vi "Dresden R2R Sputter 03.02.2018 IY24.vi"() -> ()   [LabVIEW 2009] (continued)
                                n32107 = local read "R Cmb Ch2 Step2 Coating Power Active"() -> (w36745:bool)
                                n32108 = local read "R Cmb Ch2 Step3 Coating Power Active"() -> (w36744:bool)
                                n32109 = local read "R Cmb Ch2 Step4 Coating Power Active"() -> (w36743:bool)
                                n32110 = local read "R Cmb Ch2 Step5 Coating Power Active"() -> (w36742:bool)
                                n32111 = Boolean To (0,1)(Boolean=w36746) -> (0, 1=w36741:i16)
                                n32112 = Boolean To (0,1)(Boolean=w36745) -> (0, 1=w36740:i16)
                                n32113 = Boolean To (0,1)(Boolean=w36744) -> (0, 1=w36739:i16)
                                n32114 = Boolean To (0,1)(Boolean=w36743) -> (0, 1=w36738:i16)
                                n32115 = Boolean To (0,1)(Boolean=w36742) -> (0, 1=w36737:i16)
                                n32116 = Compound Arithmetic op=ADD(w36741, w36740, w36739, w36738, w36737) -> (w36735:i16)
                                n32117 = local read "R Cmb Interval length"() -> (w36736:dbl)
                                n32118 = Wait (ms)(milliseconds to wait=u32 200) -> ()  [unwired: 1 out]
                                n32119 = Multiply(x=w36736, y=w36735) -> (x*y=w36734:dbl)
                                n32120 = local write "Total length"(w36734) -> ()
                                }
                                frame #2 {
                                n32121 = local write "Calculate 2"(TRUE ("Calculate_auto")) -> ()
                                }
                                frame #3 {
                                n32122 = local write "Roll_side_select"(enum32{"Left to Right", "Right to Left"}."Left to Right" ("Roll_side_select")) -> ()
                                }
                                frame #4 {
                                n32123 = Wait (ms)(milliseconds to wait=u32 100) -> ()  [unwired: 1 out]
                                n32124 = local write "Parameters_auto_set"(TRUE ("Parameters_auto_set")) -> ()
                                }
                                frame #5 {
                                n32125 = while {
                                i -> [w36755]
                                stop <- w36751 stop-if-true
                                n32126 = Wait Until Next ms Multiple(millisecond multiple=u32 300) -> ()  [unwired: 1 out]
                                n32127 = Greater?(x=w36755, y=100) -> (0:w36752:bool)
                                n32128 = local read "Parameters_auto_set"() -> (w36756:bool)
                                n32129 = case shown="True" w36756 {
                                tunnel: [TRUE FALSE] -> w36753
                                frame #0 {
                                }
                                frame #1 {
                                }
                                }
                                n32130 = Or(x=w36753, y=w36752) -> (x .or. y?=w36751:bool)
                                }
                                }
                                frame #6 {
                                n32131 = local read "R Tension Value"() -> (w36760:dbl)
                                n32132 = Wait (ms)(milliseconds to wait=u32 200) -> ()  [unwired: 1 out]
                                n32133 = local write "TC1_set_value"(w36760) -> ()
                                }
                                frame #7 {
                                n32134 = local write "TC1_auto_set"(TRUE ("TC1_auto_set")) -> ()
                                }
                                frame #8 {
                                w36764 = u16 2 items=["1", "2", "3", "4"] ("Target Chamber Sensor")
                                n32135 = local write "Target Chamber Sensor"(w36764) -> ()
                                n32136 = Wait (ms)(milliseconds to wait=u32 200) -> ()  [unwired: 1 out]
                                }
                                frame #9 {
                                n32137 = local read "Total length"() -> (w36765:dbl)
                                n32138 = local write "Region"(w36765) -> ()
                                }
                                frame #10 {
                                n32139 = local read "Semi"() -> (w36766:bool)
                                n32140 = case shown="False" w36766 {
                                frame #0 {
                                n32141 = stacked-sequence {
                                frame #0 {
                                # "Gas Flow"
                                n32142 = stacked-sequence {
                                frame #0 {
                                n32143 = local read "Semi"() -> (w36767:bool)
                                n32144 = case shown="False" w36767 {
                                frame #0 {
                                n32145 = stacked-sequence {
                                frame #0 {
                                n32146 = local read "Semi"() -> (w36768:bool)
                                n32147 = case shown="False" w36768 {
                                frame #0 {
                                n32148 = local read "R Argon Flow sccm"() -> (w36769:dbl)
                                n32149 = local write "Ar_sccm3_4"(w36769) -> ()
                                }
                                frame #1 {
                                }
                                }
                                }
                                frame #1 {
                                n32150 = local read "Semi"() -> (w36770:bool)
                                n32151 = case shown="False" w36770 {
                                frame #0 {
                                n32152 = local write "Mfc2_Ar _3_4_set"(TRUE ("Mfc_Ar _1_2_set")) -> ()
                                }
                                frame #1 {
                                }
                                }
                                }
                                frame #2 {
                                n32153 = local read "Semi"() -> (w36772:bool)
                                n32154 = case shown="False" w36772 {
                                frame #0 {
                                n32155 = while {
                                i -> [w36775]
                                stop <- w36777 stop-if-true
                                n32156 = Greater?(x=w36775, y=50) -> (0:w36774:bool)
                                n32157 = local read "Semi"() -> (w36773:bool)
                                n32158 = Or(x=w36773, y=w36774) -> (x .or. y?=w36777:bool)
                                }
                                }
                                frame #1 {
                                }
                                }
                                }
                                frame #3 {
                                n32159 = local read "Semi"() -> (w36778:bool)
                                n32160 = case shown="False" w36778 {
                                frame #0 {
                                n32161 = local read "Ar_sccm_act 2"() -> (w36779:dbl)
                                n32162 = Greater?(x=w36779, y=1) -> (0:w36780:bool)
                                n32163 = case shown="False" w36780 {
                                frame #0 {
                                n32164 = local read "R Argon Flow sccm"() -> (w36782:dbl)
                                n32165 = local write "Ar_sccm3_4"(w36782) -> ()
                                }
                                frame #1 {
                                }
                                }
                                }
                                frame #1 {
                                }
                                }
                                }
                                frame #4 {
                                n32166 = local read "Semi"() -> (w36783:bool)
                                n32167 = case shown="False" w36783 {
                                frame #0 {
                                n32168 = local read "Ar_sccm_act 2"() -> (w36784:dbl)
                                n32169 = Greater?(x=w36784, y=1) -> (0:w36785:bool)
                                n32170 = case shown="False" w36785 {
                                frame #0 {
                                n32171 = while {
                                i -> [w36788]
                                stop <- w36792 stop-if-true
                                n32172 = Greater?(x=w36788, y=50) -> (0:w36787:bool)
                                n32173 = local read "Semi"() -> (w36791:bool)
                                n32174 = case shown="False" w36791 {
                                tunnel: [FALSE TRUE] -> w36790
                                frame #0 {
                                n32175 = Wait Until Next ms Multiple(millisecond multiple=u32 200) -> ()  [unwired: 1 out]
                                }
                                frame #1 {
                                }
                                }
                                n32176 = Or(x=w36790, y=w36787) -> (x .or. y?=w36792:bool)
                                }
                                }
                                frame #1 {
                                }
                                }
                                }
                                frame #1 {
                                }
                                }
                                }
                                frame #5 {
                                n32177 = local read "Semi"() -> (w36796:bool)
                                n32178 = case shown="False" w36796 {
                                frame #0 {
                                n32179 = local read "Ar_sccm_act 2"() -> (w36797:dbl)
                                n32180 = Greater?(x=w36797, y=1) -> (0:w36798:bool)
                                n32181 = case shown="False" w36798 {
                                frame #0 {
                                n32182 = local write "Semi"(TRUE ("Semi")) -> ()
                                n32183 = local write "Error Message"("Coating process cancelled.\nPlease check connections." ("Error Message")) -> ()
                                }
                                frame #1 {
                                }
                                }
                                }
                                frame #1 {
                                }
                                }
                                }
                                }
                                }
                                frame #1 {
                                }
                                }
                                }
                                frame #1 {
                                n32184 = local read "Semi"() -> (w36802:bool)
                                n32185 = case shown="False" w36802 {
                                frame #0 {
                                n32186 = local write "SDC1 11"(TRUE ("SDC1 11")) -> ()
                                n32187 = Wait (ms)(milliseconds to wait=u32 1000) -> ()  [unwired: 1 out]
                                }
                                frame #1 {
                                }
                                }
                                }
                                }
                                }
                                frame #1 {
                                # "Set Pressure for ignite plasma"
                                n32188 = stacked-sequence {
                                frame #0 {
                                n32189 = local read "Semi"() -> (w36805:bool)
                                n32190 = case shown="False" w36805 {
                                frame #0 {
                                n32191 = stacked-sequence {
                                frame #0 {
                                n32192 = local read "Semi"() -> (w36806:bool)
                                n32193 = case shown="False" w36806 {
                                frame #0 {
                                n32194 = local write "Set_pressure_value 3"(10.0 ("Set_pressure_value 2")) -> ()
                                }
                                frame #1 {
                                }
                                }
                                }
                                frame #1 {
                                n32195 = local read "Semi"() -> (w36808:bool)
                                n32196 = case shown="False" w36808 {
                                frame #0 {
                                n32197 = Wait (ms)(milliseconds to wait=u32 1000) -> ()  [unwired: 1 out]
                                }
                                frame #1 {
                                }
                                }
                                }
                                frame #2 {
                                n32198 = local read "Semi"() -> (w36810:bool)
                                n32199 = case shown="False" w36810 {
                                frame #0 {
                                n32200 = local write "Pc_bv3_auto_set_pressure"(TRUE ("Pc_bv1_auto_set_pressure")) -> ()
                                }
                                frame #1 {
                                }
                                }
                                }
                                frame #3 {
                                n32201 = local read "Semi"() -> (w36812:bool)
                                n32202 = case shown="False" w36812 {
                                frame #0 {
                                n32203 = while {
                                i -> [w36823]
                                stop <- w36815 stop-if-true
                                w36813 = 10.0 ("Set_pressure_value 2")
                                n32204 = Greater?(x=w36823, y=300) -> (0:w36817:bool)
                                n32205 = Add(x=1.0, y=w36813) -> (x+y=w36819:dbl)
                                n32206 = Subtract(x=w36813, y=1.0) -> (x-y=w36820:dbl)
                                n32207 = local read "Pressure_ch3"() -> (w36814:i32)
                                n32208 = In Range and Coerce(upper limit=w36819, x=w36814, lower limit=w36820) -> (In Range?=w36818:bool)  [unwired: 1 out]
                                n32209 = case shown="False" w36818 {
                                tunnel: [FALSE TRUE] -> w36816
                                frame #0 {
                                n32210 = Wait Until Next ms Multiple(millisecond multiple=u32 200) -> ()  [unwired: 1 out]
                                }
                                frame #1 {
                                }
                                }
                                n32211 = Or(x=w36816, y=w36817) -> (x .or. y?=w36815:bool)
                                }
                                }
                                frame #1 {
                                }
                                }
                                }
                                frame #4 {
                                n32212 = local read "Semi"() -> (w36828:bool)
                                n32213 = case shown="False" w36828 {
                                frame #0 {
                                w36829 = 10.0 ("Set_pressure_value 2")
                                n32214 = Add(x=1.0, y=w36829) -> (x+y=w36832:dbl)
                                n32215 = Subtract(x=w36829, y=1.0) -> (x-y=w36833:dbl)
                                n32216 = local read "Pressure_ch3"() -> (w36830:i32)
                                n32217 = In Range and Coerce(upper limit=w36832, x=w36830, lower limit=w36833) -> (In Range?=w36831:bool)  [unwired: 1 out]
                                n32218 = case shown="False" w36831 {
                                frame #0 {
                                n32219 = local read "R Set Pressure mtorr"() -> (w36836:dbl)
                                n32220 = local write "Set_pressure_value 3"(w36836) -> ()
                                }
                                frame #1 {
                                }
                                }
                                }
                                frame #1 {
                                }
                                }
                                }
                                frame #5 {
                                n32221 = local read "Semi"() -> (w36837:bool)
                                n32222 = case shown="False" w36837 {
                                frame #0 {
                                w36838 = 10.0 ("Set_pressure_value 2")
                                n32223 = Add(x=1.0, y=w36838) -> (x+y=w36841:dbl)
                                n32224 = Subtract(x=w36838, y=1.0) -> (x-y=w36842:dbl)
                                n32225 = local read "Pressure_ch3"() -> (w36839:i32)
                                n32226 = In Range and Coerce(upper limit=w36841, x=w36839, lower limit=w36842) -> (In Range?=w36840:bool)  [unwired: 1 out]
                                n32227 = case shown="False" w36840 {
                                frame #0 {
                                n32228 = local write "Pc_bv3_auto_set_pressure"(TRUE ("Pc_bv1_auto_set_pressure")) -> ()
                                }
                                frame #1 {
                                }
                                }
                                }
                                frame #1 {
                                }
                                }
                                }
                                frame #6 {
                                n32229 = local read "Semi"() -> (w36846:bool)
                                n32230 = case shown="False" w36846 {
                                frame #0 {
                                n32231 = while {
                                i -> [w36857]
                                stop <- w36849 stop-if-true
                                w36847 = 10.0 ("Set_pressure_value 2")
                                n32232 = Greater?(x=w36857, y=300) -> (0:w36851:bool)
                                n32233 = Add(x=1.0, y=w36847) -> (x+y=w36853:dbl)
                                n32234 = Subtract(x=w36847, y=1.0) -> (x-y=w36854:dbl)
                                n32235 = local read "Pressure_ch3"() -> (w36848:i32)
                                n32236 = In Range and Coerce(upper limit=w36853, x=w36848, lower limit=w36854) -> (In Range?=w36852:bool)  [unwired: 1 out]
                                n32237 = case shown="False" w36852 {
                                tunnel: [FALSE TRUE] -> w36850
                                frame #0 {
                                n32238 = Wait Until Next ms Multiple(millisecond multiple=u32 200) -> ()  [unwired: 1 out]
                                }
                                frame #1 {
                                }
                                }
                                n32239 = Or(x=w36850, y=w36851) -> (x .or. y?=w36849:bool)
                                }
                                }
                                frame #1 {
                                }
                                }
                                }
                                frame #7 {
                                n32240 = local read "Semi"() -> (w36862:bool)
                                n32241 = case shown="False" w36862 {
                                frame #0 {
                                n32242 = local read "Set_pressure_value 3"() -> (w36865:dbl)
                                n32243 = Add(x=1.0, y=w36865) -> (x+y=w36866:dbl)
                                n32244 = Subtract(x=w36865, y=1.0) -> (x-y=w36867:dbl)
                                n32245 = local read "Pressure_ch3"() -> (w36863:i32)
                                n32246 = In Range and Coerce(upper limit=w36866, x=w36863, lower limit=w36867) -> (In Range?=w36864:bool)  [unwired: 1 out]
                                n32247 = case shown="False" w36864 {
                                frame #0 {
                                n32248 = local write "Semi"(TRUE ("Semi")) -> ()
                                n32249 = local write "Error Message"("Coating Pressure could not be adjusted !" ("Error Message")) -> ()
                                }
                                frame #1 {
                                }
                                }
                                }
                                frame #1 {
                                }
                                }
                                }
                                }
                                }
                                frame #1 {
                                }
                                }
                                }
                                frame #1 {
                                n32250 = local read "Semi"() -> (w36872:bool)
                                n32251 = case shown="False" w36872 {
                                frame #0 {
                                n32252 = local write "SDC1 9"(TRUE ("SDC1 9")) -> ()
                                n32253 = Wait (ms)(milliseconds to wait=u32 1000) -> ()  [unwired: 1 out]
                                }
                                frame #1 {
                                }
                                }
                                }
                                }
                                }
                                frame #2 {
                                # "Plasma ignite and check"
                                n32254 = stacked-sequence {
                                frame #0 {
                                n32255 = local read "Semi"() -> (w36875:bool)
                                n32256 = case shown="False" w36875 {
                                frame #0 {
                                n32257 = local write "Dc_auto_on"(TRUE ("Dc_auto_on")) -> ()
                                }
                                frame #1 {
                                }
                                }
                                }
                                frame #1 {
                                n32258 = local read "Semi"() -> (w36877:bool)
                                n32259 = case shown="False" w36877 {
                                frame #0 {
                                n32260 = while {
                                i -> [w36887]
                                stop <- w36878 stop-if-true
                                n32261 = Greater Or Equal?(x=w36887, y=240) -> (x >= y?=w36886:bool)
                                n32262 = case shown="True" w36886 {
                                frame #0 {
                                }
                                frame #1 {
                                n32263 = local write "Semi"(TRUE ("Semi")) -> ()
                                }
                                }
                                n32264 = local read "Set DC Power       : 2"() -> (w36883:dbl)
                                n32265 = local read "Actual DC Power : 2"() -> (w36882:dbl)
                                n32266 = Subtract(x=w36883, y=w36882) -> (x-y=w36885:dbl)
                                n32267 = Less?(x=w36885, y=10.0) -> (x < y?=w36880:bool)
                                n32268 = local read "Semi"() -> (w36879:bool)
                                n32269 = Or(x=w36880, y=w36879) -> (x .or. y?=w36878:bool)
                                n32270 = Wait Until Next ms Multiple(millisecond multiple=u32 500) -> ()  [unwired: 1 out]
                                }
                                }
                                frame #1 {
                                }
                                }
                                }
                                }
                                }
                                frame #3 {
                                # "Set Pressure for coating"
                                n32271 = stacked-sequence {
                                frame #0 {
                                n32272 = local read "Semi"() -> (w36890:bool)
                                n32273 = case shown="False" w36890 {
                                frame #0 {
                                n32274 = stacked-sequence {
                                frame #0 {
                                n32275 = local read "Semi"() -> (w36891:bool)
                                n32276 = case shown="False" w36891 {
                                frame #0 {
                                n32277 = local read "R Set Pressure mtorr"() -> (w36892:dbl)
                                n32278 = local write "Set_pressure_value 3"(w36892) -> ()
                                }
                                frame #1 {
                                }
                                }
                                }
                                frame #1 {
                                n32279 = local read "Semi"() -> (w36893:bool)
                                n32280 = case shown="False" w36893 {
                                frame #0 {
                                n32281 = Wait (ms)(milliseconds to wait=u32 200) -> ()  [unwired: 1 out]
                                }
                                frame #1 {
                                }
                                }
                                }
                                frame #2 {
                                n32282 = local read "Semi"() -> (w36895:bool)
                                n32283 = case shown="False" w36895 {
                                frame #0 {
                                n32284 = local write "Pc_bv3_auto_set_pressure"(TRUE ("Pc_bv1_auto_set_pressure")) -> ()
                                }
                                frame #1 {
                                }
                                }
                                }
                                frame #3 {
                                n32285 = local read "Semi"() -> (w36897:bool)
                                n32286 = case shown="False" w36897 {
                                frame #0 {
                                n32287 = while {
                                i -> [w36908]
                                stop <- w36900 stop-if-true
                                n32288 = local read "Set_pressure_value 3"() -> (w36898:dbl)
                                n32289 = Greater?(x=w36908, y=300) -> (0:w36902:bool)
                                n32290 = Add(x=1.0, y=w36898) -> (x+y=w36904:dbl)
                                n32291 = Subtract(x=w36898, y=1.0) -> (x-y=w36905:dbl)
                                n32292 = local read "Pressure_ch3"() -> (w36899:i32)
                                n32293 = In Range and Coerce(upper limit=w36904, x=w36899, lower limit=w36905) -> (In Range?=w36903:bool)  [unwired: 1 out]
                                n32294 = case shown="False" w36903 {
                                tunnel: [FALSE TRUE] -> w36901
                                frame #0 {
                                n32295 = Wait Until Next ms Multiple(millisecond multiple=u32 200) -> ()  [unwired: 1 out]
                                }
                                frame #1 {
                                }
                                }
                                n32296 = Or(x=w36901, y=w36902) -> (x .or. y?=w36900:bool)
                                }
                                }
                                frame #1 {
                                }
                                }
                                }
                                frame #4 {
                                n32297 = local read "Semi"() -> (w36913:bool)
                                n32298 = case shown="False" w36913 {
                                frame #0 {
                                n32299 = local read "Set_pressure_value 3"() -> (w36914:dbl)
                                n32300 = Add(x=1.0, y=w36914) -> (x+y=w36917:dbl)
                                n32301 = Subtract(x=w36914, y=1.0) -> (x-y=w36918:dbl)
                                n32302 = local read "Pressure_ch3"() -> (w36915:i32)
                                n32303 = In Range and Coerce(upper limit=w36917, x=w36915, lower limit=w36918) -> (In Range?=w36916:bool)  [unwired: 1 out]
                                n32304 = case shown="False" w36916 {
                                frame #0 {
                                n32305 = local read "R Set Pressure mtorr"() -> (w36921:dbl)
                                n32306 = local write "Set_pressure_value 3"(w36921) -> ()
                                }
                                frame #1 {
                                }
                                }
                                }
                                frame #1 {
                                }
                                }
                                }
                                frame #5 {
                                n32307 = local read "Semi"() -> (w36922:bool)
                                n32308 = case shown="False" w36922 {
                                frame #0 {
                                n32309 = local read "Set_pressure_value 3"() -> (w36923:dbl)
                                n32310 = Add(x=1.0, y=w36923) -> (x+y=w36926:dbl)
                                n32311 = Subtract(x=w36923, y=1.0) -> (x-y=w36927:dbl)
                                n32312 = local read "Pressure_ch3"() -> (w36924:i32)
                                n32313 = In Range and Coerce(upper limit=w36926, x=w36924, lower limit=w36927) -> (In Range?=w36925:bool)  [unwired: 1 out]
                                n32314 = case shown="False" w36925 {
                                frame #0 {
                                n32315 = local write "Pc_bv3_auto_set_pressure"(TRUE ("Pc_bv1_auto_set_pressure")) -> ()
                                }
                                frame #1 {
                                }
                                }
                                }
                                frame #1 {
                                }
                                }
                                }
                                frame #6 {
                                n32316 = local read "Semi"() -> (w36931:bool)
                                n32317 = case shown="False" w36931 {
                                frame #0 {
                                n32318 = while {
                                i -> [w36942]
                                stop <- w36933 stop-if-true
                                n32319 = local read "Set_pressure_value 3"() -> (w36937:dbl)
                                n32320 = Greater?(x=w36942, y=300) -> (0:w36935:bool)
                                n32321 = Add(x=1.0, y=w36937) -> (x+y=w36938:dbl)
                                n32322 = Subtract(x=w36937, y=1.0) -> (x-y=w36939:dbl)
                                n32323 = local read "Pressure_ch3"() -> (w36932:i32)
                                n32324 = In Range and Coerce(upper limit=w36938, x=w36932, lower limit=w36939) -> (In Range?=w36936:bool)  [unwired: 1 out]
                                n32325 = case shown="False" w36936 {
                                tunnel: [FALSE TRUE] -> w36934
                                frame #0 {
                                n32326 = Wait Until Next ms Multiple(millisecond multiple=u32 200) -> ()  [unwired: 1 out]
                                }
                                frame #1 {
                                }
                                }
                                n32327 = Or(x=w36934, y=w36935) -> (x .or. y?=w36933:bool)
                                }
                                }
                                frame #1 {
                                }
                                }
                                }
                                frame #7 {
                                n32328 = local read "Semi"() -> (w36947:bool)
                                n32329 = case shown="False" w36947 {
                                frame #0 {
                                n32330 = local read "Set_pressure_value 3"() -> (w36950:dbl)
                                n32331 = Add(x=1.0, y=w36950) -> (x+y=w36951:dbl)
                                n32332 = Subtract(x=w36950, y=1.0) -> (x-y=w36952:dbl)
                                n32333 = local read "Pressure_ch3"() -> (w36948:i32)
                                n32334 = In Range and Coerce(upper limit=w36951, x=w36948, lower limit=w36952) -> (In Range?=w36949:bool)  [unwired: 1 out]
                                n32335 = case shown="False" w36949 {
                                frame #0 {
                                n32336 = local write "Semi"(TRUE ("Semi")) -> ()
                                n32337 = local write "Error Message"("Coating Pressure could not be adjusted !" ("Error Message")) -> ()
                                }
                                frame #1 {
                                }
                                }
                                }
                                frame #1 {
                                }
                                }
                                }
                                }
                                }
                                frame #1 {
                                }
                                }
                                }
                                frame #1 {
                                n32338 = local read "Semi"() -> (w36957:bool)
                                n32339 = case shown="False" w36957 {
                                frame #0 {
                                n32340 = local write "SDC1 9"(TRUE ("SDC1 9")) -> ()
                                n32341 = Wait (ms)(milliseconds to wait=u32 1000) -> ()  [unwired: 1 out]
                                }
                                frame #1 {
                                }
                                }
                                }
                                }
                                }
                                }
                                }
                                frame #1 {
                                }
                                }
                                }
                                frame #11 {
                                n32342 = local read "Semi"() -> (w36960:bool)
                                n32343 = case shown="False" w36960 {
                                frame #0 {
                                n32344 = local write "Start_roll"(TRUE ("Start_roll")) -> ()
                                n32345 = Wait (ms)(milliseconds to wait=u32 300) -> ()  [unwired: 1 out]
                                }
                                frame #1 {
                                }
                                }
                                }
                                frame #12 {
                                n32346 = local read "Semi"() -> (w36963:bool)
                                n32347 = case shown="False" w36963 {
                                frame #0 {
                                n32348 = stacked-sequence {
                                frame #0 {
                                n32349 = local read "R Cmb Ch2 Step1 Coating Power Active"() -> (w36964:bool)
                                n32350 = case shown="True" w36964 {
                                frame #0 {
                                }
                                frame #1 {
                                n32351 = while {
                                stop <- w36966 stop-if-true
                                n32352 = local read "R Cmb Interval length"() -> (w36970:dbl)
                                n32353 = local read "Actual Length"() -> (w36969:dbl)
                                n32354 = Greater Or Equal?(x=w36969, y=w36970) -> (x >= y?=w36968:bool)
                                n32355 = local read "Semi"() -> (w36967:bool)
                                n32356 = Or(x=w36968, y=w36967) -> (x .or. y?=w36966:bool)
                                n32357 = Wait Until Next ms Multiple(millisecond multiple=u32 300) -> ()  [unwired: 1 out]
                                }
                                }
                                }
                                }
                                frame #1 {
                                n32358 = local read "R Cmb Ch2 Step2 Coating Power Active"() -> (w36971:bool)
                                n32359 = case shown="True" w36971 {
                                frame #0 {
                                }
                                frame #1 {
                                n32360 = stacked-sequence {
                                frame #0 {
                                n32361 = local read "Semi"() -> (w36972:bool)
                                n32362 = case shown="False" w36972 {
                                frame #0 {
                                n32363 = local read "R Cmb Ch3 Step2 Coating Power"() -> (w36974:dbl)
                                n32364 = Wait (ms)(milliseconds to wait=u32 200) -> ()  [unwired: 1 out]
                                n32365 = local write "Set DC Power       : 2"(w36974) -> ()
                                }
                                frame #1 {
                                }
                                }
                                }
                                frame #1 {
                                n32366 = local read "Semi"() -> (w36975:bool)
                                n32367 = case shown="False" w36975 {
                                frame #0 {
                                n32368 = local write "Dc_auto_set"(TRUE ("Dc_auto_set")) -> ()
                                }
                                frame #1 {
                                }
                                }
                                }
                                frame #2 {
                                n32369 = while {
                                stop <- w36981 stop-if-true
                                n32370 = local read "R Cmb Interval length"() -> (w36980:dbl)
                                n32371 = local read "Actual Length"() -> (w36984:dbl)
                                n32372 = Multiply(x=w36980, y=2.0) -> (x*y=w36978:dbl)
                                n32373 = Greater Or Equal?(x=w36984, y=w36978) -> (x >= y?=w36983:bool)
                                n32374 = local read "Semi"() -> (w36982:bool)
                                n32375 = Or(x=w36983, y=w36982) -> (x .or. y?=w36981:bool)
                                n32376 = Wait Until Next ms Multiple(millisecond multiple=u32 300) -> ()  [unwired: 1 out]
                                }
                                }
                                }
                                }
                                }
                                }
                                frame #2 {
                                n32377 = local read "R Cmb Ch2 Step3 Coating Power Active"() -> (w36985:bool)
                                n32378 = case shown="True" w36985 {
                                frame #0 {
                                }
                                frame #1 {
                                n32379 = stacked-sequence {
                                frame #0 {
                                n32380 = local read "Semi"() -> (w36986:bool)
                                n32381 = case shown="False" w36986 {
                                frame #0 {
                                n32382 = local read "R Cmb Ch3 Step3 Coating Power"() -> (w36988:dbl)
                                n32383 = Wait (ms)(milliseconds to wait=u32 200) -> ()  [unwired: 1 out]
                                n32384 = local write "Set DC Power       : 2"(w36988) -> ()
                                }
                                frame #1 {
                                }
                                }
                                }
                                frame #1 {
                                n32385 = local read "Semi"() -> (w36989:bool)
                                n32386 = case shown="False" w36989 {
                                frame #0 {
                                n32387 = local write "Dc_auto_set"(TRUE ("Dc_auto_set")) -> ()
                                }
                                frame #1 {
                                }
                                }
                                }
                                frame #2 {
                                n32388 = while {
                                stop <- w36995 stop-if-true
                                n32389 = local read "R Cmb Interval length"() -> (w36994:dbl)
                                n32390 = local read "Actual Length"() -> (w36998:dbl)
                                n32391 = Multiply(x=w36994, y=3.0) -> (x*y=w36992:dbl)
                                n32392 = Greater Or Equal?(x=w36998, y=w36992) -> (x >= y?=w36997:bool)
                                n32393 = local read "Semi"() -> (w36996:bool)
                                n32394 = Or(x=w36997, y=w36996) -> (x .or. y?=w36995:bool)
                                n32395 = Wait Until Next ms Multiple(millisecond multiple=u32 300) -> ()  [unwired: 1 out]
                                }
                                }
                                }
                                }
                                }
                                }
                                frame #3 {
                                n32396 = local read "R Cmb Ch2 Step4 Coating Power Active"() -> (w36999:bool)
                                n32397 = case shown="True" w36999 {
                                frame #0 {
                                }
                                frame #1 {
                                n32398 = stacked-sequence {
                                frame #0 {
                                n32399 = local read "Semi"() -> (w37000:bool)
                                n32400 = case shown="False" w37000 {
                                frame #0 {
                                n32401 = local read "R Cmb Ch3 Step4 Coating Power"() -> (w37002:dbl)
                                n32402 = Wait (ms)(milliseconds to wait=u32 200) -> ()  [unwired: 1 out]
                                n32403 = local write "Set DC Power       : 2"(w37002) -> ()
                                }
                                frame #1 {
                                }
                                }
                                }
                                frame #1 {
                                n32404 = local read "Semi"() -> (w37003:bool)
                                n32405 = case shown="False" w37003 {
                                frame #0 {
                                n32406 = local write "Dc_auto_set"(TRUE ("Dc_auto_set")) -> ()
                                }
                                frame #1 {
                                }
                                }
                                }
                                frame #2 {
                                n32407 = while {
                                stop <- w37009 stop-if-true
                                n32408 = local read "R Cmb Interval length"() -> (w37008:dbl)
                                n32409 = local read "Actual Length"() -> (w37012:dbl)
                                n32410 = Multiply(x=w37008, y=4.0) -> (x*y=w37006:dbl)
                                n32411 = Greater Or Equal?(x=w37012, y=w37006) -> (x >= y?=w37011:bool)
                                n32412 = local read "Semi"() -> (w37010:bool)
                                n32413 = Or(x=w37011, y=w37010) -> (x .or. y?=w37009:bool)
                                n32414 = Wait Until Next ms Multiple(millisecond multiple=u32 300) -> ()  [unwired: 1 out]
                                }
                                }